vi "UHR-Fleezers Control (host) - 10.0.vi"() -> ()   [LabVIEW 2009] (continued)
        n622 = To Single Precision Float(number=w1638) -> (single precision float=w1644:sgl[][])
        n623 = To Single Precision Float(number=w1640) -> (single precision float=w1641:sgl[][])
        n624 = call "IMAQ ArrayToImage"("Image Pixels (Float)"=w1672, "Image"=w1606) -> ("Image Out"=w1675:T2)  [unwired: 8 in, 1 out]
        n625 = call "IMAQ ArrayToImage"("Image Pixels (Float)"=w1613, "Image"=w1605) -> ("Image Out"=w1615:T2)  [unwired: 8 in, 1 out]
        n626 = call "IMAQ ArrayToImage"("Image Pixels (Float)"=w1644, "Image"=w1604) -> ("Image Out"=w1646:T2)  [unwired: 8 in, 1 out]
        n627 = call "IMAQ ArrayToImage"("Image Pixels (Float)"=w1641, "Image"=w1603) -> ("Image Out"=w1643:T2)  [unwired: 8 in, 1 out]
        n628 = call "IMAQ Symmetry"("Type of Symmetry"=w1674, "Image Src"=w1675) -> ("Image Dst Out"=w1670:T2)  [unwired: 3 in, 1 out]
        n629 = call "IMAQ Symmetry"("Type of Symmetry"=w1614, "Image Src"=w1615) -> ("Image Dst Out"=w1611:T2)  [unwired: 3 in, 1 out]
        n630 = call "IMAQ Symmetry"("Type of Symmetry"=w1645, "Image Src"=w1646) -> ("Image Dst Out"=→"Detection Laser X":T2)  [unwired: 3 in, 1 out]
        n631 = call "IMAQ Symmetry"("Type of Symmetry"=w1642, "Image Src"=w1643) -> ("Image Dst Out"=→"Detection Laser Y":T2)  [unwired: 3 in, 1 out]
        n632 = call "IMAQ Set Simple Calibration"("Calibration Axis Info"=T26 {"Origin Pixel"={"X"=0.0, "Y"=0.0}, "Angle Relative to Horizontal (deg)"=0.0, "Axis Reference"=0}, "Grid Descriptor"=T27 {"X Step"=0.3, "Y Step"=0.3, "Unit"=enum."Undefined"}, "Image"=w1670) -> ("Calibrated Image"=→"APD 1":T2)  [unwired: 7 in, 1 out]
        n633 = call "IMAQ Set Simple Calibration"("Calibration Axis Info"=T26 {"Origin Pixel"={"X"=0.0, "Y"=0.0}, "Angle Relative to Horizontal (deg)"=0.0, "Axis Reference"=0}, "Grid Descriptor"=T27 {"X Step"=0.3, "Y Step"=0.3, "Unit"=enum."Undefined"}, "Image"=w1611) -> ("Calibrated Image"=→"APD 2":T2)  [unwired: 7 in, 1 out]
      }
    }
    n634 = Subtract(x=w780, y="APD 2 Offset") -> (x-y=w777:waveform(dbl))
    n635 = Subtract(x=w782, y="APD 1 Offset") -> (x-y=w778:waveform(dbl))
    n636 = Index Array(array=w797, index=3) -> (element=w872:waveform(dbl))
    n637 = Index Array(array=w797, index=6) -> (element=w869:waveform(dbl))
    n638 = Build Array(w778, w777) -> (→"APD Chart":waveform(dbl)[])
    n639 = Array Size(array=w861) -> (size(s)=w916:i32)
    n640 = call <vilib>:"Std Deviation and Variance.vi"("X"=w790) -> ("standard deviation"=w789:dbl)  [unwired: 1 in, 2 out]
    n641 = Add Array Elements(numeric array=w790) -> (sum=w792:u32)
    n642 = Add Array Elements(numeric array=w861) -> (sum=w926:u32)
    n643 = call <vilib>:"Std Deviation and Variance.vi"("X"=w861) -> ("standard deviation"=w860:dbl)  [unwired: 1 in, 2 out]
    n644 = Divide(x="T1 offset_x (mV)", y=1000.0) -> (x/y=w873:dbl)
    n645 = Divide(x=w789, y=w788) -> (x/y=w785:dbl)
    "Rate sigma (Hz) 2" <- w785
    n646 = Multiply(x=w788, y=w916) -> (x*y=w791:dbl)
    "Int. Time (s)" <- w791
    n647 = Divide(x=w792, y=w791) -> (x/y=w786:dbl)
    "APD 2 Rate (Hz)" <- w786
    n648 = Divide(x=w926, y=w791) -> (x/y=w858:dbl)
    "APD 1 Rate (Hz)" <- w858
    n649 = Divide(x=w860, y=w788) -> (x/y=w859:dbl)
    "Rate sigma (Hz)" <- w859
    n650 = Divide(x=w785, y=w786) -> (x/y=→"Sigma/Mean 2":dbl)
    n651 = Divide(x=w859, y=w858) -> (x/y=→"Sigma/Mean":dbl)
    n652 = Divide(x="T2 offset_x (mV)", y=1000.0) -> (x/y=w871:dbl)
    n653 = case shown="0, Default" "Calibration" {
      tunnel: "T1 alpha_x (nm/V)" -> [_ w1569 w1590]
      tunnel: "T1 kappa_x (pN/nm)" -> [_ _ w1580]
      tunnel: "T2 alpha_x (nm/V)" -> [_ w1568 w1588]
      tunnel: "T2 kappa_x (pN/nm)" -> [_ _ w1581]
      tunnel: w872 -> [w1551 w1566 w1586]
      tunnel: w869 -> [w1550 w1564 w1584]
      tunnel: [w1551 w1563 w1583] -> w902
      tunnel: [w1550 w1562 w1582] -> w901
      tunnel: ["T1 X (V)" ("Label.Text") "T1 X (nm)" ("Label.Text") "T1 X (pN)" ("Label.Text")] -> w890
      tunnel: ["T2 X (V)" ("Label.Text") "T2 X (nm)" ("Label.Text") "T2 X (pN)" ("Label.Text")] -> w889
      tunnel: ["Position (V)" ("Label.Text") "Position (nm)" ("Label.Text") "Force (pN)" ("Label.Text")] -> w891
      tunnel: w871 -> [_ w1554 w1573]
      tunnel: w873 -> [_ w1557 w1575]
      tunnel: ["Mean (V)" ("Label.Text") "Mean (nm)" ("Label.Text") "Mean (pN)" ("Label.Text")] -> w886
      tunnel: ["Difference (V)" ("Label.Text") "Difference (nm)" ("Label.Text") "Difference (pN)" ("Label.Text")] -> w805
      frame #0 {
      }
      frame #1 {
        n654 = Unbundle By Name(w1566) -> ("Y"=w1570:dbl[])
        n655 = Unbundle By Name(w1564) -> ("Y"=w1555:dbl[])
        n656 = Subtract(x=w1570, y=w1557) -> (x-y=w1558:dbl[])
        n657 = Subtract(x=w1555, y=w1554) -> (x-y=w1556:dbl[])
        n658 = Multiply(x=w1556, y=w1568) -> (x*y=w1565:dbl[])
        n659 = Multiply(x=w1569, y=w1558) -> (x*y=w1567:dbl[])
        n660 = Bundle By Name(cluster=w1564, "Y"=w1565) -> (w1562:waveform(dbl))
        n661 = Bundle By Name(cluster=w1566, "Y"=w1567) -> (w1563:waveform(dbl))
      }
      frame #2 {
        n662 = Unbundle By Name(w1586) -> ("Y"=w1591:dbl[])
        n663 = Unbundle By Name(w1584) -> ("Y"=w1589:dbl[])
        n664 = Subtract(x=w1589, y=w1573) -> (x-y=w1574:dbl[])
        n665 = Subtract(x=w1591, y=w1575) -> (x-y=w1576:dbl[])
        n666 = Compound Arithmetic op=MULTIPLY(w1574, w1588, w1581) -> (w1585:dbl[])
        n667 = Compound Arithmetic op=MULTIPLY(w1580, w1590, w1576) -> (w1587:dbl[])
        n668 = Bundle By Name(cluster=w1584, "Y"=w1585) -> (w1582:waveform(dbl))
        n669 = Bundle By Name(cluster=w1586, "Y"=w1587) -> (w1583:waveform(dbl))
      }
    }
    n670 = feedback #16(u16 1 ("Calibration")) -> (w893:u16)
    n671 = Not Equal?(x=w893, y="Calibration") -> (x != y?=w846:bool)
    n672 = Unbundle By Name(w872) -> ("Y"=w875:dbl[])
    n673 = Unbundle By Name(w869) -> ("Y"=w878:dbl[])
    n674 = Subtract(x=w875, y=w873) -> (x-y=w876:dbl[])
    n675 = Subtract(x=w878, y=w871) -> (x-y=w877:dbl[])
    n676 = Multiply(x=w877, y="T2 alpha_x (nm/V)") -> (x*y=w868:dbl[])
    n677 = Multiply(x="T1 alpha_x (nm/V)", y=w876) -> (x*y=w867:dbl[])
    n678 = Multiply(x=w901, y=-1.0) -> (x*y=w880:waveform(dbl))
    n679 = case shown="True" "Read Lateness and Rel Phase" {
      tunnel: w842 -> [w1194 w1214]
      tunnel: w841 -> [w1195 w1213]
      tunnel: [w1194 w1212] -> w864
      tunnel: [w1195 w1211] -> w863
      frame #0 {
      }
      frame #1 {
        n680 = xnode "Read/Write Control"("FPGA VI Reference In"=w1214, "error in"=w1213) -> ("FPGA VI Reference Out"=w1212:T20, "error out"=w1211:errorcluster, "GI Relative phase"=→"GI relative phase":i16, "Relative phase"=→"Relative phase (AI1)":i16, "AI Late Counter"=→"Late Counter (AI1)":u32, "GI Late Counter"=→"GI Late Counter":u32, "MCL Late Counter"=→"MCL Late Counter":u32, "MCL Relative Phase"=→"Relative Phase (MCL)":i16, "APD Acq Relative Phase"=→"APD Acq Relative Phase":i16, "APD 1 Gate Relative Phase"=→"APD 1 Gate Relative Phase":i16, "APD 2 Gate Relative Phase"=→"APD 2 Gate Relative Phase":i16, "APD Acq Late Counter"=→"APD Acq Late Counter":u32, "APD 1 Gate Late Counter"=→"APD 1 Gate Late Counter":u32, "APD 2 Gate Late Counter"=→"APD 2 Gate Late Counter":u32, "Green FB Relative Phase"=→"Relative phase (Green FB)":i16, "GI Relative phase 2"=→"GI relative phase 2":i16, "GI Late Counter 2"=→"GI Late Counter 2":u32)
      }
    }
    n681 = Subtract(x=w868, y=w867) -> (x-y=w866:dbl[])
    n682 = Unbundle By Name(w901) -> ("Y"=w831:dbl[])
    n683 = Unbundle By Name(w902) -> ("Y"=w832:dbl[])
    n684 = Build Array(w902, w880) -> (→"Force":waveform(dbl)[])
    n685 = Subtract(x=w866, y="Offset (nm)") -> (x-y=w829:dbl[])
    n686 = call <vilib>:"Mean.vi"("X"=w831) -> ("mean"=w809:dbl)  [unwired: 1 out]
    "T2 X" <- w809
    n687 = Absolute Value(x=w832) -> (abs(x)=w833:dbl[])
    n688 = Absolute Value(x=w831) -> (abs(x)=w834:dbl[])
    n689 = call <vilib>:"Mean.vi"("X"=w832) -> ("mean"=w810:dbl)  [unwired: 1 out]
    "T1 X" <- w810
    n690 = Add(x=w833, y=w834) -> (x+y=w835:dbl[])
    n691 = Bundle By Name(cluster=w872, "Y"=w829) -> (w796:waveform(dbl))
    "Bead Separation" <- w796
    n692 = Divide(x=w835, y=2.0) -> (x/y=→"Vec Mean of T1 T2":dbl[])
    n693 = case shown="True" w846 {
      tunnel: w891 -> [_ w1544]
      tunnel: w890 -> [_ w1543]
      tunnel: w889 -> [_ w1542]
      tunnel: w886 -> [_ w1541]
      tunnel: w805 -> [_ w1540]
      frame #0 {
      }
      frame #1 {
        n694 = property on="Force" class="WFChart (strict)"("YScale.NameLbl.Text"=w1544) -> ()  [unwired: 2 in, 2 out]
        n695 = property on="T2 X" class="DigNum (strict)"("Caption.Text"=w1542) -> ()  [unwired: 2 in, 2 out]
        n696 = property on="T1 X" class="DigNum (strict)"("Caption.Text"=w1543) -> ()  [unwired: 2 in, 2 out]
        n697 = property on="Mean" class="DigNum (strict)"("Caption.Text"=w1541) -> ()  [unwired: 2 in, 2 out]
        n698 = property on="Difference" class="DigNum (strict)"("Caption.Text"=w1540) -> ()  [unwired: 2 in, 2 out]
      }
    }
    n699 = local read "Tether"() -> (w838:bool)
    n700 = Absolute Value(x=w810) -> (abs(x)=w807:dbl)
    n701 = Absolute Value(x=w809) -> (abs(x)=w806:dbl)
    n702 = local read "Display Period (s)"() -> (w824:dbl)
    n703 = Add(x=w807, y=w806) -> (x+y=w888:dbl)
    n704 = Subtract(x=w807, y=w806) -> (x-y=→"Difference":dbl)
    n705 = feedback #17(w829) -> (w828:dbl[])
    n706 = Divide(x=w888, y=2.0) -> (x/y=w837:dbl)
    "Mean" <- w837
    n707 = case shown="True" w838 {
      tunnel: w837 -> [_ w1154]
      frame #0 {
      }
      frame #1 {
        n708 = Greater?(x="Lost Tether Alarm Threshold (pN)", y=w1154) -> (0:w1152:bool)
        n709 = case shown="True" w1152 {
          frame #0 {
          }
          frame #1 {
            n710 = flat-sequence {
              frame #0 {
                # "stop only if saving"
                n711 = local read "Saving..."() -> (w1166:bool)
                n712 = And(x=w1166, y="TA Cancel Save?") -> (x .and. y?=w1165:bool)
                n713 = local write "Stop Saving"(w1165) -> ()
              }
              frame #1 {
                n714 = case shown="True" "TA Green Off?" {
                  frame #0 {
                  }
                  frame #1 {
                    w1169 = FALSE ("Fl. Triggered...")
                    n715 = local write "Fl. Triggered..."(w1169) -> ()
                    n716 = property on="Green Laser ON/Interlacing" class="Bool (strict)"("Val(Sgnl)"=w1169) -> ()  [unwired: 2 in, 2 out]
                  }
                }
              }
            }
            n717 = local read "Time tether formed"() -> (w1160:timestamp)
            n718 = Get Date/Time In Seconds() -> (seconds since 1Jan1904=w1161:timestamp)
            n719 = Subtract(x=w1161, y=w1160) -> (x-y=w1159:dbl)
            n720 = Number To Decimal String(number=w1159) -> (decimal integer string=w1156:string)  [unwired: 1 out]
            n721 = local read "Messages"() -> (w1163:string)
            n722 = call <vilib>:"Beep.vi"() -> ()  [unwired: 3 in, 9 out]
            n723 = Concatenate Strings("Lost tether (" ("Message to add"), w1156, " s)." ("string")) -> (w1158:string)
            n724 = local write "Tether"(FALSE ("Tether")) -> ()
            n725 = call "Update messages.vi"("Message to add"=w1158, "Old message string"=w1163) -> ("New message string"=w1162:string)
            n726 = local write "Messages"(w1162) -> ()
          }
        }
      }
    }
    n727 = Build Array (concatenate)(w829, w828) -> (w827:dbl[])
    n728 = Divide(x="Bead Sep. Int. Time (s)", y=w824) -> (x/y=w823:dbl)
    n729 = Split 1D Array(array=w827, index=w823) -> (first subarray=w822:dbl[])  [unwired: 1 out]
    n730 = call <vilib>:"Mean.vi"("X"=w822) -> ("mean"=w821:dbl)  [unwired: 1 out]
    "Bead Mean (nm)" <- w821
    n731 = Subtract(x=w822, y=w821) -> (x-y=w820:dbl[])
    n732 = Square(x=w820) -> (x^2=w819:dbl[])
    n733 = call <vilib>:"Mean.vi"("X"=w819) -> ("mean"=w818:dbl)  [unwired: 1 out]
    n734 = Square Root(x=w818) -> (sqrt(x)=w817:dbl)
    n735 = Multiply(x=10.0, y=w817) -> (x*y=→"RMS (Ang)":dbl)
    n736 = xnode "Read/Write Control"("FPGA VI Reference In"=w864, "error in"=w863) -> ("FPGA VI Reference Out"=w985:T20, "error out"=w979:errorcluster, "AI2 Y Sum Set 1"=w975:i16, "AI2 Y Sum Set 2"=w974:i16, "AI1 X Set 1"=w736:fxp<+/-,16,1>, "AI1 X Set 2"=w735:fxp<+/-,16,1>, "Trap Pos FB Action"=w729:i64, "Scanning"=→"AOD Scanning":bool, "Scan I"=→"AOD Scan I":u64, "Scanning MCL"=w977:bool, "Scan I (MCL)"=→"MCL Scan I":u64, "Green FB Signals"=w911:T31)  [unwired: 1 out]
    "MCL Scanning" <- w977
    "Trap Pos FB Action" <- w729
    n737 = local read "AI2 (V)"() -> (w976:cluster{"Set 1":dbl, "Set 2":dbl})
    n738 = Bundle By Name(cluster=w976, "Set 1"=w975, "Set 2"=w974) -> (w972:cluster{"Set 1":dbl, "Set 2":dbl})
    n739 = Divide(x=w729, y=327.67) -> (x/y=→"Action (%)":dbl)
    n740 = local read "Trap X AI1"() -> (w751:T10)
    n741 = Divide(x=w972, y=3276.7) -> (x/y=w971:cluster{"Set 1":dbl, "Set 2":dbl})
    n742 = local write "AI2 (V)"(w971) -> ()
    n743 = Bundle(cluster=w751, "Set 1"=w736, "Set 2"=w735) -> (→"Trap X AI1":T10)
    n744 = Divide(x=w911, y=3276.7) -> (x/y=w907:T39)
    n745 = Unbundle By Name(w907) -> ("Green FB Ch 0"=w910:dbl, "Green FB Ch 1"=w909:dbl, "Green FB Ch 2"=w908:dbl)
    n746 = Divide(x=w910, y=w908) -> (x/y=w906:dbl)
    n747 = Divide(x=w909, y=w908) -> (x/y=w905:dbl)
    n748 = flat-sequence "To save data" {
      tunnel: [w3681] -> w997
      tunnel: [w3682] -> w996
      tunnel: w942 -> [w3675]
      tunnel: w825 -> [w3679]
      tunnel: ["Save Calibration"] -> w967
      tunnel: w962 -> [w3678]
      tunnel: [w3671] -> w961
      tunnel: [w3668] -> w960
      tunnel: [w3665] -> w959
      tunnel: w941 -> [w3667]
      tunnel: w844 -> [w3661]
      tunnel: [w3661] -> w843
      tunnel: ["Start Saving"] -> w798
      tunnel: w997 -> [w3881]
      tunnel: w996 -> [w3880]
      tunnel: w749 -> [w3879]
      tunnel: w967 -> [w3878]
      tunnel: w961 -> [w3876]
      tunnel: w960 -> [w3875]
      tunnel: w959 -> [w3874]
      tunnel: w811 -> [w3873]
      tunnel: w856 -> [w3872]
      tunnel: w843 -> [w3871]
      tunnel: w798 -> [w3870]
      tunnel: w796 -> [w3869]
      tunnel: w772 -> [w3868]
      frame #0 {
        n749 = Or(x="Save N Sets", y="Start Saving") -> (x .or. y?=w3662:bool)
        n750 = To Double Precision Float(number=w3678) -> (double precision float=w3672:dbl)
        n751 = Build Array(w3662, "Save Calibration", w3675, w3667) -> (w3677:bool[])
        n752 = Compound Arithmetic op=OR("Save Calibration", w3675, w3662, w3667) -> (w3680:bool)
        n753 = Boolean Array To Number(Boolean array=w3677) -> (number=w3674:u32)
        n754 = feedback #18(refnum<k0> refnum) -> (w3683:refnum<file>)
        n755 = feedback #19(FALSE ("Save APD Data\nwith Trap Data")) -> (w3666:bool)
        n756 = feedback #20(refnum<k0> refnum) -> (w3669:refnum<file>)
        n757 = feedback #21(0) -> (w3685:i32)
        n758 = feedback #22() -> (w3673:u32)  [unwired: 1 out]
        n759 = case shown="True" w3680 {
          tunnel: [w3690 1] -> w3681
          tunnel: w3685 -> [w3692 _]
          tunnel: [w3691 w3705] -> w3682
          tunnel: w3683 -> [w3691 _]
          tunnel: w3679 -> [_ w3725]
          tunnel: w3672 -> [_ w3723]
          tunnel: w3674 -> [_ w3726]
          tunnel: [w3689 w3704] -> w3671
          tunnel: w3673 -> [w3689 _]
          tunnel: [w3688 w3701] -> w3668
          tunnel: w3669 -> [w3688 _]
          tunnel: [w3687 w3700] -> w3665
          tunnel: w3666 -> [w3687 _]
          tunnel: "Start Saving" -> [_ w3698]
          tunnel: w3661 -> [_ w3697]
          frame #0 {
            n760 = Increment(x=w3692) -> (x+1=w3690:i32)
          }
          frame #1 {
            w3693 = FALSE ("Start Saving")
            w3699 = 9.0  # File Version
            w3708 = FALSE ("prepend array or string size? (T)")
            w3706 = T33."big-endian, network order" ("byte order (0:big-endian, network order)")
            n761 = Array Size(array=w3697) -> (size(s)=w3696:i32)
            n762 = local read "BD 1 Frequency 1 (MHz)"() -> (w3722:dbl)
            n763 = local read "BD 2 Frequency 1 (MHz)"() -> (w3721:dbl)
            n764 = local read "BD 1 Frequency 2 (MHz)"() -> (w3720:dbl)
            n765 = local read "BD 2 Frequency 2 (MHz)"() -> (w3719:dbl)
            n766 = local read "BD 1 Frequency 3 (MHz)"() -> (w3718:dbl)
            n767 = local read "BD 2 Frequency 3 (MHz)"() -> (w3717:dbl)
            n768 = To Double Precision Float(number=w3696) -> (double precision float=w3695:dbl)
            n769 = local write "Save Calibration"(w3693) -> ()
            n770 = local write "Start Saving"(w3693) -> ()
            n771 = Build Array(w3722, w3721, w3720, w3719, w3718, w3717) -> (w3716:dbl[])
            n772 = case shown="1, Default" w3726 {
              tunnel: w3725 -> [w3774 w3794 w3809 w3846]
              tunnel: w3695 -> [w3779 w3801 w3829 w3865]
              tunnel: w3723 -> [w3778 w3800 w3828 w3864]
              tunnel: [w3775 w3796 w3820 w3856] -> w3714
              tunnel: [w3765 "Cal sets to save" w3810 w3847] -> w3704
              tunnel: w3716 -> [w3776 w3797 w3822 w3858]
              tunnel: "Save APD Data\nwith Trap Data" -> [w3773 _ w3805 w3843]
              tunnel: [w3773 w3790 w3805 w3843] -> w3700
              tunnel: w3699 -> [w3768 w3788 w3803 w3841]
              tunnel: w3698 -> [w3767 _ _ _]
              frame #0 {
                # "timeseries"
                n773 = case shown="True" "Profile" {
                  tunnel: [w3782 w3786] -> w3762
                  tunnel: [w3782 w3785] -> w3761
                  tunnel: [w3782 w3784] -> w3760
                  tunnel: [w3782 w3783] -> w3759
                  frame #0 {
                    w3782 = 0.0 ("f")
                  }
                  frame #1 {
                    n774 = local read "Current Position"() -> (w3787:cluster{dbl, dbl, dbl})
                    n775 = local read "Y change (mm)"() -> (w3783:dbl)
                    n776 = Unbundle(w3787) -> (w3786:dbl, w3785:dbl, w3784:dbl)
                  }
                }
                n777 = local read "Save ave N"() -> (w3781:dbl)
                n778 = Multiply(x=w3781, y=w3774) -> (x*y=w3780:dbl)
                n779 = Boolean To (0,1)(Boolean=w3773) -> (0, 1=w3772:i16)
                n780 = To Double Precision Float(number=w3772) -> (double precision float=w3771:dbl)
                n781 = Build Array(w3768, w3774, w3780, w3779, w3778, 0.0 ("f")) -> (w3777:dbl[])
                n782 = Build Array(w3771, w3762, w3761, w3760, w3759) -> (w3769:dbl[])
                n783 = Select(t=u32 4000000000, s=w3767, f="N sets to save") -> (s? t:f=w3765:u32)
                n784 = Build Array (concatenate)(w3777, w3776, w3769) -> (w3775:dbl[])
              }
              frame #1 {
                w3791 = 0.0 ("f")
                w3790 = FALSE ("Save APD Data\nwith Trap Data")
                # "calibration"
                n785 = Boolean To (0,1)(Boolean=w3790) -> (0, 1=w3793:i16)
                n786 = To Double Precision Float(number=w3793) -> (double precision float=w3792:dbl)
                n787 = Build Array(w3792, w3791, w3791, w3791, w3791) -> (w3789:dbl[])
                n788 = Build Array(w3788, w3794, w3794, w3801, w3800, 1.0 ("t")) -> (w3798:dbl[])
                n789 = Build Array (concatenate)(w3798, w3797, w3789) -> (w3796:dbl[])
                "Calibrating Trap..." <- TRUE ("Calibrating...")
              }
              frame #2 {
                w3806 = 0.0 ("f")
                # "scan dir (x/y = 0/1)"
                # "cycles/step"
                # "n scans (f/b)"
                # "steps"
                # "freq. range"
                # "AOD raster scan"
                n790 = local read "Number of F/B Scans (AOD)"() -> (w3814:u16)
                n791 = local read "Cycles/step (AOD)"() -> (w3816:u64)
                n792 = local read "Scan Range (MHz)"() -> (w3819:dbl)
                n793 = local read "Scan steps (AOD)"() -> (w3818:u64)
                n794 = local read "Scan BD"() -> (w3826:bool)
                n795 = local read "Save ave N"() -> (w3831:dbl)
                n796 = Boolean To (0,1)(Boolean=w3826) -> (0, 1=w3825:i16)
                n797 = To Double Precision Float(number=w3814) -> (double precision float=w3813:dbl)
                n798 = To Double Precision Float(number=w3818) -> (double precision float=w3817:dbl)
                n799 = To Double Precision Float(number=w3816) -> (double precision float=w3815:dbl)
                n800 = To Double Precision Float(number=w3825) -> (double precision float=w3824:dbl)
                n801 = Boolean To (0,1)(Boolean=w3805) -> (0, 1=w3808:i16)
                n802 = Multiply(x=w3831, y=w3809) -> (x*y=w3830:dbl)
                n803 = To Double Precision Float(number=w3808) -> (double precision float=w3807:dbl)
                n804 = Build Array(w3807, w3806, w3806, w3806, w3806) -> (w3804:dbl[])
                n805 = local read "N sets should be saved"() -> (w3811:dbl)
                n806 = Build Array(w3824, w3819, w3817, w3815, w3813) -> (w3821:dbl[])
                n807 = Build Array(w3803, w3809, w3830, w3829, w3828, 2.0 ("t")) -> (w3823:dbl[])
                n808 = Round Toward +Infinity(x=w3811) -> (ceil(x): smallest int >= x=w3812:dbl)
                n809 = Build Array (concatenate)(w3823, w3822, w3804, w3821) -> (w3820:dbl[])
                n810 = To Unsigned Long Integer(number=w3812) -> (unsigned 32bit integer=w3810:u32)
              }
              frame #3 {
                w3838 = 0.0 ("f")
                # "MCL raster scan"
                n811 = local read "Number of scans (MCL)"() -> (w3833:u64)
                n812 = local read "Scan lines (y)"() -> (w3832:u64)
                n813 = local read "2D or 1D Scan"() -> (w3835:bool)
                n814 = local read "Scan Range (V)\n(of steps)"() -> (w3855:dbl)
                n815 = local read "Fast Scan Dir"() -> (w3862:bool)
                n816 = local read "Cycles/step (MCL)"() -> (w3852:u64)
                n817 = local read "Scan steps (MCL)"() -> (w3854:u64)
                n818 = Select(t=w3832, s=w3835, f=w3833) -> (s? t:f=w3834:u64)
                n819 = Boolean To (0,1)(Boolean=w3835) -> (0, 1=w3837:i16)
                n820 = local read "Save ave N"() -> (w3867:dbl)
                n821 = local read "Initial X"() -> (w3840:dbl)
                n822 = local read "Initial Y"() -> (w3839:dbl)
                n823 = To Double Precision Float(number=w3837) -> (double precision float=w3836:dbl)
                n824 = Boolean To (0,1)(Boolean=w3862) -> (0, 1=w3861:i16)
                n825 = To Double Precision Float(number=w3834) -> (double precision float=w3850:dbl)
                n826 = To Double Precision Float(number=w3854) -> (double precision float=w3853:dbl)
                n827 = To Double Precision Float(number=w3852) -> (double precision float=w3851:dbl)
                n828 = To Double Precision Float(number=w3861) -> (double precision float=w3860:dbl)
                n829 = Boolean To (0,1)(Boolean=w3843) -> (0, 1=w3845:i16)
                n830 = Multiply(x=w3867, y=w3846) -> (x*y=w3866:dbl)
                n831 = To Double Precision Float(number=w3845) -> (double precision float=w3844:dbl)
                n832 = local read "N sets should be saved (MCL)"() -> (w3848:dbl)
                n833 = Build Array(w3844, w3836, w3838, w3838, w3838) -> (w3842:dbl[])
                n834 = Build Array(w3860, w3855, w3853, w3851, w3850, w3840, w3839) -> (w3857:dbl[])
                n835 = Build Array(w3841, w3846, w3866, w3865, w3864, 3.0 ("t")) -> (w3859:dbl[])
                n836 = Round Toward +Infinity(x=w3848) -> (ceil(x): smallest int >= x=w3849:dbl)
                n837 = Build Array (concatenate)(w3859, w3858, w3842, w3857) -> (w3856:dbl[])
                n838 = To Unsigned Long Integer(number=w3849) -> (unsigned 32bit integer=w3847:u32)
              }
            }
            n839 = local read "Index"() -> (w3731:dbl)
            n840 = call "Create new save file.vi"("Insert"="", "Ext"=".dat", "Index In"=w3731) -> ("Path Out"=w3702:path, "Index Out"=w3703:dbl)
            n841 = local write "Save file name"(w3702) -> ()
            n842 = local write "Index"(w3703) -> ()
            n843 = local write "Save index"(w3703) -> ()
            n844 = Array Size(array=w3714) -> (size(s)=w3715:i32)
            n845 = Open/Create/Replace File(file path (use dialog)=w3702, operation (0:open)=T32."create", access (0:read/write)=enum16{"read/write", "read-only", "write-only"}."write-only") -> (refnum out=w3728:refnum<file>)  [unwired: 1 in, 4 out]
            n846 = local write "Saving..."(TRUE ("Saving...")) -> ()
            n847 = To Double Precision Float(number=w3715) -> (double precision float=w3713:dbl)
            n848 = String Length(string="Comment (data description)") -> (length=w3711:i32)
            n849 = To Double Precision Float(number=w3711) -> (double precision float=w3710:dbl)
            n850 = Deny Access(7:w3728) -> (3:w3727:refnum<file>)  [unwired: 1 in, 2 out]
            n851 = Build Array (concatenate)(w3713, w3714, w3710) -> (w3712:dbl[])
            n852 = case "If fluorescence data to be saved" shown="True" w3700 {
              tunnel: w3702 -> [_ w3758]
              tunnel: [refnum<k0> refnum w3738] -> w3701
              frame #0 {
              }
              frame #1 {
                w3737 = 0.0
                n853 = local read "APD Integration Time (s)"() -> (w3743:dbl)
                n854 = local read "N APD Samp/step"() -> (w3736:dbl)
                n855 = Path To String(path=w3758) -> (string=w3757:string)
                n856 = String Length(string=w3757) -> (length=w3756:i32)
                n857 = Subtract(x=w3756, y=4) -> (x-y=w3754:i32)
                n858 = String Subset(string=w3757, length (rest)=w3754) -> (substring=w3753:string)  [unwired: 1 out]
                n859 = Build Array(w3743, w3736, w3737, w3737, w3737, w3737, w3737, w3737) -> (w3740:dbl[])
                n860 = Concatenate Strings(w3753, "_fl.dat" ("string")) -> (w3751:string)
                n861 = Array Size(array=w3740) -> (size(s)=w3742:i32)
                n862 = String To Path(string=w3751) -> (path=w3747:path)
                n863 = Open/Create/Replace File(file path (use dialog)=w3747, operation (0:open)=T32."create", access (0:read/write)=enum16{"read/write", "read-only", "write-only"}."write-only") -> (refnum out=w3748:refnum<file>)  [unwired: 1 in, 4 out]
                n864 = Deny Access(7:w3748) -> (3:w3744:refnum<file>)  [unwired: 1 in, 2 out]
                n865 = To Double Precision Float(number=w3742) -> (double precision float=w3741:dbl)
                n866 = Build Array (concatenate)(w3741, w3740) -> (w3739:dbl[])
                n867 = Write to Binary File(file (use dialog)=w3744, data=w3739, 5:FALSE ("prepend array or string size? (T)"), 9:T33."big-endian, network order" ("byte order (0:big-endian, network order)")) -> (refnum out=w3738:refnum<file>)  [unwired: 1 in, 3 out]
              }
            }
            n868 = Write to Binary File(file (use dialog)=w3727, data=w3712, 5:w3708, 9:w3706) -> (refnum out=w3709:refnum<file>)  [unwired: 1 in, 3 out]
            n869 = Write to Binary File(file (use dialog)=w3709, data="Comment (data description)", 5:w3708, 9:w3706) -> (refnum out=w3705:refnum<file>)  [unwired: 1 in, 3 out]
          }
        }
      }
      frame #1 {
        n870 = local read "Saving..."() -> (w3877:bool)
        n871 = case shown="True" w3877 {
          tunnel: w3881 -> [_ w3888]
          tunnel: w3880 -> [_ w3902]
          tunnel: w3879 -> [_ w3898]
          tunnel: w3878 -> [_ w3897]
          tunnel: w3876 -> [_ w3896]
          tunnel: w3875 -> [_ w3891]
          tunnel: w3874 -> [_ w3890]
          tunnel: w3873 -> [_ w3889]
          tunnel: w3872 -> [_ w3887]
          tunnel: w3871 -> [_ w3885]
          tunnel: w3870 -> [_ w3884]
          tunnel: w3869 -> [_ w3883]
          tunnel: w3868 -> [_ w3882]
          frame #0 {
          }
          frame #1 {
            n872 = Multiply(x=w3888, y=w3887) -> (x*y=→"Time (s)":dbl)
            n873 = Less Or Equal?(x=w3888, y=w3896) -> (x <= y?=w3900:bool)
            n874 = Or(x="Stop Saving", y="Abort save 2") -> (x .or. y?=w3892:bool)
            n875 = Not(x=w3892) -> (.not. x?=w3901:bool)
            n876 = And(x=w3900, y=w3901) -> (x .and. y?=w3899:bool)
            n877 = case shown="True" w3899 {
              tunnel: w3902 -> [w3907 w3970]
              tunnel: [0.0 w3973] -> w3895
              tunnel: w3888 -> [_ w3971]
              tunnel: w3896 -> [_ w3972]
              tunnel: w3898 -> [_ w3967]
              tunnel: w3897 -> [_ _]
              tunnel: w3891 -> [w3905 w3958]
              tunnel: w3890 -> [w3904 w3959]
              tunnel: w3889 -> [_ w3957]
              tunnel: w3885 -> [_ w3956]
              tunnel: w3884 -> [_ w3910]
              tunnel: w3883 -> [_ w3949]
              tunnel: w3882 -> [_ w3927]
              frame #0 {
                w3903 = FALSE
                n878 = Close File(refnum=w3907) -> ()  [unwired: 1 in, 2 out]
                n879 = case shown="True" w3904 {
                  tunnel: w3905 -> [_ w3908]
                  frame #0 {
                  }
                  frame #1 {
                    n880 = Close File(refnum=w3908) -> ()  [unwired: 1 in, 2 out]
                  }
                }
                n881 = local write "Raster Scanning..."(w3903) -> ()
                n882 = local write "Calibrating Trap..."(w3903) -> ()
                n883 = call <vilib>:"Beep.vi"() -> ()  [unwired: 3 in, 9 out]
                n884 = local write "Stop Saving"(w3903) -> ()
                "Saving..." <- w3903
              }
              frame #1 {
                n885 = local read "Calibrating Trap..."() -> (w3960:bool)
                n886 = case shown="True" w3959 {
                  tunnel: w3958 -> [_ w3977]
                  tunnel: w3957 -> [_ w3976]
                  frame #0 {
                  }
                  frame #1 {
                    n887 = Write to Binary File(file (use dialog)=w3977, data=w3976, 5:FALSE ("prepend array or string size? (T)"), 9:T33."big-endian, network order" ("byte order (0:big-endian, network order)")) -> ()  [unwired: 1 in, 4 out]
                  }
                }
                n888 = Greater?(x="Save ave N", y=1.0) -> (0:w3963:bool)
                n889 = Not(x=w3960) -> (.not. x?=w3962:bool)
                n890 = And(x=w3962, y=w3963) -> (x .and. y?=w3964:bool)
                n891 = case shown="True" w3964 {
                  tunnel: w3967 -> [w3980 w3992]
                  tunnel: [w3980 w3984] -> w3961
                  tunnel: "Save ave N" -> [_ w3985]
                  tunnel: w3956 -> [_ w3983]
                  frame #0 {
                  }
                  frame #1 {
                    n892 = Array Size(array=w3992) -> (size(s)=w3986:i32)
                    n893 = Array Size(array=w3983) -> (size(s)=w3982:i32)
                    n894 = Divide(x=w3986, y=w3982) -> (x/y=w3990:dbl)
                    n895 = Reshape Array(w3992, w3990, w3982) -> (w3991:i16[][])
                    n896 = Transpose 2D Array(2D array=w3991) -> (transposed array=w3989:i16[][])
                    n897 = for {
                      tunnel: w3989 -> [w3995] mode=indexing
                      tunnel: [w3994] -> w3981 mode=indexing
                      tunnel: w3985 -> [w3993]
                      workers-P: _ -> [_]
                      n898 = call "downsample 1D array - I16.vi"("Ave N"=w3993, "Array In"=w3995) -> ("Array Out"=w3994:i16[])  [unwired: 1 out]
                    }
                    n899 = Transpose 2D Array(2D array=w3981) -> (transposed array=w3988:i16[][])
                    n900 = Divide(x=w3986, y=w3985) -> (x/y=w3987:dbl)
                    n901 = Reshape Array(w3988, w3987) -> (w3984:i16[])
                  }
                }
                n902 = Index Array(array=w3927, index=1) -> (element=w3930:waveform(dbl))
                n903 = Index Array(array=w3927, index=0) -> (element=w3932:waveform(dbl))
                n904 = Unbundle By Name(w3930) -> ("Y"=w3934:dbl[])
                n905 = Unbundle By Name(w3932) -> ("Y"=w3942:dbl[])
                n906 = Write to Binary File(file (use dialog)=w3970, data=w3961, 5:FALSE ("prepend array or string size? (T)"), 9:T33."big-endian, network order" ("byte order (0:big-endian, network order)")) -> ()  [unwired: 1 in, 4 out]
                n907 = feedback #23(w3934) -> (w3936:dbl[])
                n908 = Build Array (concatenate)(w3936, w3934) -> (w3935:dbl[])
                n909 = Select(t=w3934, s=w3910, f=w3935) -> (s? t:f=w3920:dbl[])
                n910 = feedback #24(w3942) -> (w3955:dbl[])
                n911 = Build Array (concatenate)(w3955, w3942) -> (w3954:dbl[])
                n912 = Select(t=w3942, s=w3910, f=w3954) -> (s? t:f=w3929:dbl[])
                n913 = Divide(x=w3971, y=w3972) -> (x/y=w3974:dbl)
                n914 = Multiply(x=w3974, y=100.0) -> (x*y=w3973:dbl)
                n915 = Build Array(w3929, w3920) -> (→"Saved APD":dbl[][])
                n916 = Array Size(array=w3929) -> (size(s)=w3947:i32)
                n917 = Unbundle By Name(w3949) -> ("Y"=w3953:dbl[])
                n918 = Subtract(x=w3947, y="N pts to average") -> (x-y=w3923:i32)
                n919 = Multiply(x="N pts to average", y=u16 2) -> (x*y=w3924:u16)
                n920 = Subtract(x=w3947, y=w3924) -> (x-y=w3922:i32)
                n921 = feedback #25(w3953) -> (w3952:dbl[])
                n922 = Build Array (concatenate)(w3952, w3953) -> (w3951:dbl[])
                n923 = Select(t=w3953, s=w3910, f=w3951) -> (s? t:f=w3950:dbl[])
                "Trap Delta Graph" <- w3950
                n924 = Array Subset(array=w3929, index=w3923, length="N pts to average") -> (w3946:dbl[])
                n925 = Array Subset(array=w3929, index=w3922, length="N pts to average") -> (w3945:dbl[])
                n926 = Array Subset(array=w3920, index=w3923, length="N pts to average") -> (w3926:dbl[])
                n927 = Array Subset(array=w3920, index=w3922, length="N pts to average") -> (w3925:dbl[])
                n928 = call <vilib>:"Mean.vi"("X"=w3946) -> ("mean"=w3944:dbl)  [unwired: 1 out]
                n929 = call <vilib>:"Mean.vi"("X"=w3926) -> ("mean"=w3919:dbl)  [unwired: 1 out]
                n930 = call <vilib>:"Mean.vi"("X"=w3945) -> ("mean"=w3943:dbl)  [unwired: 1 out]
                n931 = call <vilib>:"Mean.vi"("X"=w3925) -> ("mean"=w3918:dbl)  [unwired: 1 out]
                n932 = Subtract(x=w3919, y=w3918) -> (x-y=w3909:dbl)
                "Delta Fl. 2" <- w3909
                n933 = Subtract(x=w3944, y=w3943) -> (x-y=w3941:dbl)
                "Delta Fl. 1" <- w3941
                n934 = Initialize Array(w3941, 1 ("dimension size")) -> (w3938:dbl[])
                n935 = Initialize Array(w3909, 1 ("dimension size")) -> (w3915:dbl[])
                n936 = feedback #26(w3938) -> (w3939:dbl[])
                n937 = Build Array (concatenate)(w3939, w3938) -> (w3937:dbl[])
                n938 = feedback #27(w3915) -> (w3916:dbl[])
                n939 = Build Array (concatenate)(w3916, w3915) -> (w3914:dbl[])
                n940 = Select(t=w3938, s=w3910, f=w3937) -> (s? t:f=w3913:dbl[])
                n941 = Select(t=w3915, s=w3910, f=w3914) -> (s? t:f=w3912:dbl[])
                n942 = Build Array(w3913, w3912) -> (→"Save APD Deriv":dbl[][])
              }
            }
            "Progress" <- w3895
            "Progress 2" <- w3895
          }
        }
      }
    }
    n943 = Bundle By Name(cluster=w907, "Green FB Ch 0"=w906, "Green FB Ch 1"=w905) -> (w885:T39)
    "Green FB Signals (V)" <- w885
    n944 = Unbundle By Name(w885) -> ("Green FB Ch 2"=→"Green FB Plot":dbl)
    n945 = local read "wait to reset values"() -> (w980:bool)
    n946 = Not(x=w977) -> (.not. x?=w981:bool)
    n947 = And(x=w981, y=w980) -> (x .and. y?=w982:bool)
    n948 = case "Part of MCL raster scanning: returns to initial positions after scan done" shown="True" w982 {
      tunnel: w985 -> [w2491 w2498]
      tunnel: [w2491 w2497] -> w984
      tunnel: w979 -> [w2490 w2496]
      tunnel: [w2490 w2495] -> w978
      frame #0 {
      }
      frame #1 {
        w2506 = 10.0 ("y")
        w2505 = 32767.0 ("y")
        # "to return scan values\nafter a synchronous \nAOM scan"
        n949 = local read "AO2"() -> (w2499:dbl)
        n950 = local read "AO1"() -> (w2500:dbl)
        n951 = Multiply(x=w2500, y=w2505) -> (x*y=w2502:dbl)
        n952 = local write "wait to reset values"(FALSE ("wait to reset values")) -> ()
        n953 = Multiply(x=w2499, y=w2505) -> (x*y=w2504:dbl)
        n954 = Divide(x=w2502, y=w2506) -> (x/y=w2501:dbl)
        n955 = Divide(x=w2504, y=w2506) -> (x/y=w2503:dbl)
        n956 = To Word Integer(number=w2501) -> (16bit integer=w2507:i16)
        n957 = To Word Integer(number=w2503) -> (16bit integer=w2508:i16)
        n958 = local read "Total Counts (ticks)"() -> (w2492:u32)
        n959 = xnode "Read/Write Control"("FPGA VI Reference In"=w2498, "error in"=w2496, "AO1"=w2507, "AO2"=w2508, "MCL count"=w2492) -> ("FPGA VI Reference Out"=w2497:T20, "error out"=w2495:errorcluster)
        n960 = local read "Scan Range (V)\n(of steps)"() -> (w2493:dbl)
        n961 = property on="Scan Range (V)\n(of steps)" class="DigNum (strict)"("Val(Sgnl)"=w2493) -> ()  [unwired: 2 in, 2 out]
      }
    }
    n962 = node-c288() -> ()  [unwired: 2 out]
  }
  n963 = flat-sequence "Video" {
    tunnel: [w4076] -> w40
    tunnel: w40 -> [w4116]
    frame #0 {
      n964 = while {
        stop <- w4069 continue-if-true
        n965 = call "Close Video Capture.vi"() -> ("error code OUT"=w4071:i32)
        n966 = Equal?(x=w4071, y=0) -> (x = y?=w4069:bool)
      }
      n967 = local write "Stop All"(FALSE ("Stop All")) -> ()
    }
    frame #1 {
      n968 = call "DMR_Init.vi"() -> ()  [unwired: 3 out]
    }
    frame #2 {
      # "Setting the destination format to Mono8 makes sure that the image can be displayed in the intensity plot."
      n969 = call "DMR_GetDevice.vi"("search string IN"="DE019116701") -> ("device handle OUT"=w4094:i32)  [unwired: 4 in, 2 out]
      n970 = call "DMR_OpenDevice.vi"("device handle IN"=w4094) -> ("driver handle OUT"=w4077:i32)  [unwired: 4 out]
      n971 = call "DMR_FindList.vi"("flags IN"=u32 0 ("flags"), "list name IN"="" ("String"), "list type IN"=T40."camera descriptions", "driver handle IN"=w4077) -> ("list handle OUT"=w4080:i32)  [unwired: 2 out]
      n972 = call "DMR_FindList.vi"("flags IN"=u32 0 ("flags"), "list name IN"="Base", "list type IN"=T40."setting", "driver handle IN"=w4077) -> ("list handle OUT"=w4078:i32)  [unwired: 2 out]
      n973 = call "OBJ_GetHandle.vi"("object name IN"="VideoStandard", "list handle IN"=w4080) -> ("object handle OUT"=w4074:i32)  [unwired: 3 out]
      n974 = call "OBJ_GetHandle.vi"("object name IN"="PixelFormat", "list handle IN"=w4078) -> ("object handle OUT"=w4088:i32)  [unwired: 3 out]
      n975 = call "OBJ_SetS.vi"("value index IN"=0, "value IN"="NTSC M", "object handle IN"=w4074) -> ()  [unwired: 2 out]
      n976 = call "OBJ_SetS.vi"("value index IN"=0, "value IN"="Mono8" ("value"), "object handle IN"=w4088) -> ()  [unwired: 2 out]
      n977 = call "OBJ_GetHandle.vi"("object name IN"="VideoChannel", "list handle IN"=w4078) -> ("object handle OUT"=w4084:i32)  [unwired: 3 out]
      n978 = while {
        tunnel: [w4099] -> w4076
        tunnel: w4077 -> [w4096]
        stop <- w4097 continue-if-true
        n979 = call "DMR_ImageRequestSingle.vi"("request control IN"=0, "driver handle IN"=w4096) -> ("error code OUT"=w4098:i32, "driver handle OUT"=w4099:i32)  [unwired: 2 out]
        n980 = Equal To 0?(x=w4098) -> (x = 0?=w4097:bool)
      }
      n981 = call "OBJ_SetI.vi"("value index IN"=0, "value IN"=3 ("Video channel"), "object handle IN"=w4084) -> ()  [unwired: 2 out]
    }
    frame #3 {
      w4104 = T16 0 items=["Grayscale (U8)", "Grayscale (I16)", "Grayscale (SGL)", "Complex (CSG)", "RGB (U32)", "HSL (U32)", "RGB (U64)"] ("Image Type")
      w4112 = T16 0 items=["Grayscale (U8)", "Grayscale (I16)", "Grayscale (SGL)", "Complex (CSG)", "RGB (U32)", "HSL (U32)", "RGB (U64)"] ("Image Type")
      n982 = for "Create Greyscale map" {
        N: 256 -> [_]
        tunnel: [w4118] -> w4101 mode=indexing
        workers-P: _ -> [_]
        i -> [w4121]
        n983 = To Unsigned Byte Integer(number=w4121) -> (unsigned 8bit integer=w4117:u8)
        n984 = Join Numbers(hi=w4117, lo=w4117) -> ((hi.lo)=w4120:u16)
        n985 = Join Numbers(hi=w4117, lo=w4117) -> ((hi.lo)=w4119:u16)
        n986 = Join Numbers(hi=w4120, lo=w4119) -> ((hi.lo)=w4118:u32)
      }
      n987 = call "IMAQ Create"("Image Name"="Scaled video", "Image Type"=w4104) -> ("New Image"=w4103:T2)  [unwired: 2 in, 2 out]
      n988 = call "IMAQ Create"("Image Name"="Main video", "Image Type"=w4112) -> ("New Image"=w4113:T2)  [unwired: 2 in, 2 out]
      n989 = node-c288() -> (w4111:T22)  [unwired: 4 out]
      n990 = Initialize Array(u32 0 ("Window Number (0...15)"), 480 ("dimension size"), 640 ("dimension size")) -> (w4106:u32[][])
      n991 = timed-loop {
        tunnel: w4116 -> [w4138]
        tunnel: [w4137] -> w4115
        tunnel: w4113 -> [w4136]
        timing: w4111 -> [_]
        timing-out: [_] -> w4110
        tunnel: w4106 -> [w4125]
        tunnel: w4103 -> [w4123]
        tunnel: w4101 -> [w4122]
        stop <- w4124 stop-if-true
        # "This block performs the \nactual image capture."
        n992 = node-c288() -> ()  [unwired: 2 out]
        n993 = local read "Stop All"() -> (w4124:bool)
        n994 = Reciprocal(x="Video Capture Rate (Hz)") -> (1/x=w4128:dbl)
        n995 = Multiply(x=w4128, y=1000.0) -> (x*y=w4126:dbl)
        n996 = call "DMR_ImageRequestWaitFor.vi"("queue number IN"=0, "timeout(ms) IN"=500, "driver handle IN"=w4138) -> ("error code OUT"=w4142:i32, "request number OUT"=w4139:i32, "driver handle OUT"=w4140:i32)
        n997 = feedback #28(T41 refnum ("Avi Refnum")) -> (w4130:T41)
        n998 = case shown="True" "New Video File" {
          tunnel: [T41 refnum ("Avi Refnum") w4159] -> w4132
          tunnel: [FALSE TRUE] -> w4133
          tunnel: w4130 -> [_ w4155]
          frame #0 {
          }
          frame #1 {
            n999 = call "Create new save file.vi"("Ext"=".avi" ("string"), "Index In"="Video Index") -> ("Path Out"=w4151:path, "Index Out"=w4152:dbl)  [unwired: 1 in]
            "Path Out" <- w4151
            n1000 = Not Equal?(x=w4155, y=T41 refnum ("Avi Refnum")) -> (x != y?=w4156:bool)
            n1001 = Increment(x=w4152) -> (x+1=w4161:dbl)
            n1002 = case shown="True" w4156 {
              tunnel: w4155 -> [_ w4162]
              frame #0 {
              }
              frame #1 {
                n1003 = call "IMAQ AVI Close"("Avi Refnum"=w4162) -> ()  [unwired: 1 in, 10 out]
              }
            }
            n1004 = call "IMAQ AVI Create"("Frames Per Second"=u32 30, "AVI Path"=w4151) -> ("Avi Refnum"=w4159:T41)  [unwired: 5 in, 4 out]
            n1005 = local write "Video Index"(w4161) -> ()
          }
        }
        n1006 = Equal To 0?(x=w4142) -> (x = 0?=w4141:bool)
        n1007 = Select(t=w4132, s=w4133, f=w4130) -> (s? t:f=w4131:T41)
        n1008 = case shown="True" w4141 {
          tunnel: w4140 -> [w4163 w4188]
          tunnel: w4139 -> [_ w4187]
          tunnel: [w4163 w4184] -> w4137
          tunnel: w4136 -> [_ w4168]
          tunnel: w4125 -> [_ w4172]
          tunnel: w4131 -> [_ w4170]
          tunnel: w4123 -> [_ w4165]
          tunnel: w4122 -> [_ w4164]
          frame #0 {
          }
          frame #1 {
            w4178 = u32 0 ("X-offset IN")
            n1009 = call "DMR_GetImageRequestBufferData.vi"("driver handle IN"=w4188, "request number IN"=w4187) -> ("width OUT"=w4177:i32, "height OUT"=w4176:i32, "driver handle OUT"=w4183:i32, "request number OUT"=w4182:i32, "bytes per pixel OUT"=w4179:i32)  [unwired: 13 out]
            n1010 = call "DMR_GetImageRequestBufferImageData.vi"("driver handle IN"=w4183, "request number IN"=w4182, "bytes per pixel IN"=w4179, "X-offset IN"=w4178, "Y-offset IN"=w4178, "height IN"=w4176, "width IN"=w4177) -> ("driver handle OUT"=w4181:u32, "request number OUT"=w4180:u32, "image OUT"=w4173:u32[][])  [unwired: 10 out]
            n1011 = call "DMR_ImageRequestUnlock.vi"("request number IN"=w4180, "driver handle IN"=w4181) -> ("driver handle OUT"=w4186:i32)  [unwired: 1 in, 2 out]
            n1012 = case shown="True" "Averaging" {
              tunnel: w4173 -> [w4224 w4229]
              tunnel: [w4224 w4228] -> w4169
              tunnel: w4172 -> [_ w4226]
              frame #0 {
              }
              frame #1 {
                (unwired) 1
                w4234 = 1
                n1013 = feedback #29(w4226) -> (w4225:u32[][])
                n1014 = Add(x=w4229, y=w4225) -> (x+y=w4230:u32[][])
                n1015 = Select(t=w4226, s="Reset Averaging", f=w4230) -> (s? t:f=w4232:u32[][])
                n1016 = feedback #30(w4234) -> (w4227:i32)
                n1017 = Divide(x=w4230, y=w4227) -> (x/y=w4231:dbl[][])
                n1018 = Increment(x=w4227) -> (x+1=w4235:i32)
                n1019 = To Unsigned Long Integer(number=w4231) -> (unsigned 32bit integer=w4228:u32[][])
                n1020 = Select(t=w4234, s="Reset Averaging", f=w4235) -> (s? t:f=w4233:i32)
              }
            }
            n1021 = call "DMR_ImageRequestSingle.vi"("request control IN"=0, "driver handle IN"=w4186) -> ("driver handle OUT"=w4184:i32)  [unwired: 3 out]
            n1022 = disable-structure shown="Disabled" {
              disable-tunnel: w4169 -> [w4201 _]
              disable-tunnel: w4165 -> [w4200 _]
              frame #0 {
                n1023 = To Double Precision Float(number=w4201) -> (double precision float=w4199:dbl[][])
                n1024 = In Range and Coerce(upper limit="Intensity Upper", x=w4199, lower limit="Intensity Lower") -> (coerced(x)=w4198:dbl[][])  [unwired: 1 out]
                n1025 = Subtract(x="Intensity Upper", y="Intensity Lower") -> (x-y=w4195:dbl)
                n1026 = Subtract(x=w4198, y="Intensity Lower") -> (x-y=w4196:dbl[][])
                n1027 = Divide(x=w4196, y=w4195) -> (x/y=w4197:dbl[][])
                n1028 = Multiply(x=255.0, y=w4197) -> (x*y=w4193:dbl[][])
                n1029 = To Unsigned Byte Integer(number=w4193) -> (unsigned 8bit integer=w4202:u8[][])
                n1030 = call "IMAQ ArrayToImage"("Image Pixels (U8)"=w4202, "Image"=w4200) -> ("Image Out"=w4189:T2)  [unwired: 4 in, 5 out]
                n1031 = First Call?() -> (First Call?: T/F=w4190:bool)
                n1032 = case shown="True" w4190 {
                  tunnel: w4189 -> [w4203 w4214]
                  frame #0 {
                    n1033 = flat-sequence {
                      tunnel: w4203 -> [w4209]
                      frame #0 {
                        w4206 = FALSE ("Get/Set Status? (Set)")
                        w4205 = 0 ("Window Number (0...15)")
                        n1034 = call "IMAQ WindSize"("Get/Set Status? (Set)"=w4206, "Window Number"=w4205) -> ("Width & Height out"=→"Window Size":cluster{"Width":i32, "Height":i32})  [unwired: 4 in, 2 out]
                        n1035 = call "IMAQ WindMove"("Window Number (0...15)"=w4205, "Get/Set Status? (Set)"=w4206) -> ("Coordinates (screen)"=→"Window Position":cluster{"X Position":i32, "Y Position":i32})  [unwired: 3 in, 1 out]
                        n1036 = call "IMAQ WindDraw"("Resize to Image Size? (Y)"=FALSE, "Window Number (0...15)"=w4205, "Image"=w4209) -> ()  [unwired: 7 in, 2 out]
                      }
                      frame #1 {
                        n1037 = call "IMAQ WindZoom 2"("Center Point"="Center Point", "Zoom to Fit? (False)"=FALSE, "Zoom Factor"="Zoom Factor") -> ()  [unwired: 5 in, 4 out]
                      }
                    }
                  }
                  frame #1 {
                    n1038 = flat-sequence {
                      tunnel: w4214 -> [w4217]
                      tunnel: [w4215] -> w4213
                      tunnel: w4213 -> [w4219]
                      frame #0 {
                        w4216 = TRUE ("Resize to Image Size? (Y)")
                        w4215 = 0 ("Window Number (0...15)")
                        n1039 = call "IMAQ WindNonTearing"("Window Number"=w4215, "NonTearing? (True)"=w4216) -> ()  [unwired: 8 in, 2 out]
                        n1040 = call "IMAQ WindDraw"("Resize to Image Size? (Y)"=w4216, "Window Number (0...15)"=w4215, "Image"=w4217) -> ()  [unwired: 7 in, 2 out]
                      }
                      frame #1 {
                        n1041 = call "IMAQ WindSize"("Scrollbars? (N)"=FALSE, "Width & Height"="Initial Window Size", "Window Number"=w4219) -> ()  [unwired: 3 in, 3 out]
                        n1042 = call "IMAQ WindMove"("Window Number (0...15)"=w4219, "Coordinates (screen)"="Initial Window Position") -> ()  [unwired: 3 in, 2 out]
                      }
                    }
                  }
                }
              }
              frame #1 {
              }
            }
            n1043 = To Unsigned Byte Integer(number=w4169) -> (unsigned 8bit integer=w4167:u8[][])
            n1044 = call "IMAQ ArrayToImage"("Image Pixels (U8)"=w4167, "Image"=w4168) -> ("Image Out"=w4166:T2)  [unwired: 4 in, 5 out]
            "Primary Video Display" <- w4166
            n1045 = case shown="True" "Save Video" {
              tunnel: w4170 -> [_ w4223]
              tunnel: w4166 -> [_ w4222]
              frame #0 {
              }
              frame #1 {
                n1046 = call "IMAQ AVI Write Frame"("Image"=w4222, "Avi Refnum"=w4223) -> ()  [unwired: 2 in, 8 out]
              }
            }
            n1047 = case shown="True" "Save Image" {
              tunnel: w4167 -> [_ w4238]
              tunnel: w4164 -> [_ w4237]
              frame #0 {
              }
              frame #1 {
                n1048 = call <vilib>:"Flatten Pixmap.vi"("colors"=w4237, "8-bit pixmap"=w4238) -> ("image data"=w4244:T42)  [unwired: 4 in, 5 out]
                n1049 = call "Create new save file.vi"("Insert"="video_frame_" ("string"), "Ext"=".bmp" ("string"), "Index In"="Image Index") -> ("Path Out"=w4240:path, "Index Out"=w4245:dbl)
                n1050 = Increment(x=w4245) -> (x+1=w4239:dbl)
                n1051 = local write "Image Index"(w4239) -> ()
                n1052 = call <vilib>:"Write BMP File.vi"("image data"=w4244, "path to BMP file"=w4240) -> ()  [unwired: 1 in, 9 out]